vi "Controle_Manip_Main_GUI_WorkingBackup_211222.vi"() -> ()   [LabVIEW 2019] (continued)
                n3174 = local read "ESP 301 On?"() -> (w3865:bool)
                n3175 = case shown="True" w3865 {
                  tunnel: w3867 -> [_ w3881]
                  tunnel: w3866 -> [_ w3869]
                  frame False {
                  }
                  frame True {
                    n3176 = case shown="\"RotStage Exc Angle (°)\", Default" w3881 {
                      tunnel: [2 1 3] -> w3882
                      tunnel: [w3886 w3889 w3892] -> w3878
                      tunnel: w3869 -> [w3885 w3888 w3891]
                      frame "RotStage Det Angle (°)" {
                        n3177 = local write "RotStage Det Angle (°)"(w3885) -> ()
                        n3178 = control-ref of="RotStage Det Angle Readout (°)"() -> (w3886:refnum<vi>)
                      }
                      frame "Newport Linear Translation Stage Position (mm)" {
                        n3179 = control-ref of="Newport Linear Translation Stage Position Readout (mm)"() -> (w3889:refnum<vi>)
                        n3180 = local write "Newport Linear Translation Stage Position (mm)"(w3888) -> ()
                      }
                      frame "RotStage Exc Angle (°)", Default {
                        n3181 = local write "RotStage Exc Angle (°)"(w3891) -> ()
                        n3182 = control-ref of="RotStage Exc Angle Readout (°)"() -> (w3892:refnum<vi>)
                      }
                    }
                    n3183 = local read "Excitation Wavelength (nm)"() -> (w3874:dbl)
                    n3184 = local read "Photodiode handle out"() -> (w3876:refnum<visa-resource-name>)
                    n3185 = local read "Photodiode error out"() -> (w3875:errorcluster)
                    n3186 = local read "Photodiode Status"() -> (w3868:bool)
                    n3187 = local read "ESP 301 Error"() -> (w3883:errorcluster)
                    n3188 = control-ref of="Excitation Power (uW)"() -> (w3877:refnum<vi>)
                    n3189 = call <instrlib>:"TLPM Set Wavelength.vi"("error in (no error)"=w3875, "Wavelength (0.0)"=w3874, "instrument handle"=w3876) -> ("error out"=w3872:errorcluster, "instrument handle out"=w3873:refnum<visa-resource-name>)  [unwired: 7 in]
                    n3190 = local read "ESP 301 COM Port"() -> (w3884:refnum<visa-resource-name>)
                    n3191 = call "Go2Angle.vi"("VISA resource name"=w3884, "Photodiode"=w3873, "RotStage Det Angle Readout (°) 4"=w3878, "Excitation Power (uW) 2"=w3877, "Photodiode on?"=w3868, "Axis ESP301 / RotStage"=w3882, "ESP301 Error"=w3883, "Photodiode error"=w3872, "Position (units)"=w3869) -> ("Photodiode out"=w3870:refnum<visa-resource-name>, "VISA resource name out"=w3880:refnum<visa-resource-name>, "Photodiode"=w3871:errorcluster, "ESP301 Error out"=w3879:errorcluster)  [unwired: 3 in]
                    n3192 = local write "ESP 301 COM Port"(w3880) -> ()
                    n3193 = local write "ESP 301 Error"(w3879) -> ()
                    n3194 = local write "Photodiode handle out"(w3870) -> ()
                    n3195 = local write "Photodiode error out"(w3871) -> ()
                  }
                }
              }
            }
          }
          event "RotStage Exc Home", "RotStage Det Home", "Newport Linear Translation Stage Home": Mouse Down {
            n3196 = event-data() -> ("CtlRef"=w3896:refnum<vi>)  [unwired: 1 in, 7 out]
            n3197 = property class="Bool (strict)"(reference=w3896) -> ("Label.Text"=w3895:string)  [unwired: 1 in, 2 out]
            n3198 = case shown="\"Newport Linear Translation Stage Home\"" w3895 {
              tunnel: 0.0 -> [w3897 w3898 w3899]
              frame "RotStage Det Home", Default {
                n3199 = property on="RotStage Det Angle (°)" class="DigNum (strict)"("Val(Sgnl)"=w3897) -> ()  [unwired: 2 in, 2 out]
              }
              frame "Newport Linear Translation Stage Home" {
                n3200 = property on="Newport Linear Translation Stage Position (mm)" class="DigNum (strict)"("Val(Sgnl)"=w3898) -> ()  [unwired: 2 in, 2 out]
              }
              frame "RotStage Exc Home" {
                n3201 = property on="RotStage Exc Angle (°)" class="DigNum (strict)"("Val(Sgnl)"=w3899) -> ()  [unwired: 2 in, 2 out]
              }
            }
          }
          event "RotStage Exc Jog Backward", "RotStage Det Jog Backward", "RotStage Exc Jog Forward", "RotStage Det Jog Forward", "Newport Linear Translation Stage Jog Forward", "Newport Linear Translation Stage Jog Backward", "PZC Jog Forward", "PZC Jog Backward": Mouse Down {
            n3202 = event-data() -> ("CtlRef"=w3902:refnum<vi>)  [unwired: 1 in, 7 out]
            n3203 = property class="Bool (strict)"(reference=w3902) -> ("Label.Text"=w3900:string, "Value"=w3901:bool)  [unwired: 1 in, 2 out]
            n3204 = case shown="\"PZC Jog Backward\"" w3900 {
              tunnel: w3901 -> [_ _ _ _ _ _ _ _ _]
              frame "RotStage Det Jog Backward" {
                n3205 = local read "RotStage Det Angle Readout (°)"() -> (w3905:dbl)
                n3206 = local read "RotStage Det Angle Step (°)"() -> (w3904:dbl)
                n3207 = Subtract(x=w3905, y=w3904) -> (x-y=w3903:dbl)
                n3208 = property on="RotStage Det Angle (°)" class="DigNum (strict)"("Val(Sgnl)"=w3903) -> ()  [unwired: 2 in, 2 out]
              }
              frame "RotStage Det Jog Forward" {
                n3209 = local read "RotStage Det Angle Readout (°)"() -> (w3907:dbl)
                n3210 = local read "RotStage Det Angle Step (°)"() -> (w3908:dbl)
                n3211 = Add(x=w3907, y=w3908) -> (x+y=w3906:dbl)
                n3212 = property on="RotStage Det Angle (°)" class="DigNum (strict)"("Val(Sgnl)"=w3906) -> ()  [unwired: 2 in, 2 out]
              }
              frame "RotStage Exc Jog Forward" {
                n3213 = local read "RotStage Exc Angle Readout (°)"() -> (w3911:dbl)
                n3214 = local read "RotStage Exc Angle Step (°)"() -> (w3910:dbl)
                n3215 = Add(x=w3911, y=w3910) -> (x+y=w3909:dbl)
                n3216 = property on="RotStage Exc Angle (°)" class="DigNum (strict)"("Val(Sgnl)"=w3909) -> ()  [unwired: 2 in, 2 out]
              }
              frame "Newport Linear Translation Stage Jog Forward" {
                n3217 = local read "Newport Linear Translation Stage Position Readout (mm)"() -> (w3916:dbl)
                n3218 = local read "Newport Linear Translation Stage Step (mm)"() -> (w3915:dbl)
                n3219 = Add(x=w3916, y=w3915) -> (x+y=w3914:dbl)
                n3220 = property on="Newport Linear Translation Stage Position Readout (mm)" class="DigNum (strict)"() -> ("Maximum"=w3912:dbl)  [unwired: 2 in, 2 out]
                n3221 = Less Or Equal?(x=w3914, y=w3912) -> (x <= y?=w3913:bool)
                n3222 = case shown="True" w3913 {
                  tunnel: w3914 -> [_ w3920]
                  frame False {
                    n3223 = stacked-sequence {
                      frame #0 {
                        n3224 = property on="Newport Linear Translation Stage Position Readout (mm)" class="DigNum (strict)"("Blinking"=TRUE) -> ()  [unwired: 2 in, 2 out]
                      }
                      frame #1 {
                        n3225 = Wait (ms)(milliseconds to wait=u32 500) -> ()  [unwired: 1 out]
                      }
                      frame #2 {
                        n3226 = property on="Newport Linear Translation Stage Position Readout (mm)" class="DigNum (strict)"("Blinking"=FALSE) -> ()  [unwired: 2 in, 2 out]
                      }
                    }
                  }
                  frame True {
                    n3227 = property on="Newport Linear Translation Stage Position (mm)" class="DigNum (strict)"("Val(Sgnl)"=w3920) -> ()  [unwired: 2 in, 2 out]
                  }
                }
              }
              frame "Newport Linear Translation Stage Jog Backward" {
                n3228 = local read "Newport Linear Translation Stage Position Readout (mm)"() -> (w3925:dbl)
                n3229 = local read "Newport Linear Translation Stage Step (mm)"() -> (w3924:dbl)
                n3230 = Subtract(x=w3925, y=w3924) -> (x-y=w3922:dbl)
                n3231 = property on="Newport Linear Translation Stage Position Readout (mm)" class="DigNum (strict)"() -> ("Minimum"=w3921:dbl)  [unwired: 2 in, 2 out]
                n3232 = Greater Or Equal?(x=w3922, y=w3921) -> (x >= y?=w3923:bool)
                n3233 = case shown="False" w3923 {
                  tunnel: w3922 -> [_ w3929]
                  frame False {
                    n3234 = stacked-sequence {
                      frame #0 {
                        n3235 = property on="Newport Linear Translation Stage Position Readout (mm)" class="DigNum (strict)"("Blinking"=TRUE) -> ()  [unwired: 2 in, 2 out]
                      }
                      frame #1 {
                        n3236 = Wait (ms)(milliseconds to wait=u32 500) -> ()  [unwired: 1 out]
                      }
                      frame #2 {
                        n3237 = property on="Newport Linear Translation Stage Position Readout (mm)" class="DigNum (strict)"("Blinking"=FALSE) -> ()  [unwired: 2 in, 2 out]
                      }
                    }
                  }
                  frame True {
                    n3238 = property on="Newport Linear Translation Stage Position (mm)" class="DigNum (strict)"("Val(Sgnl)"=w3929) -> ()  [unwired: 2 in, 2 out]
                  }
                }
              }
              frame "RotStage Exc Jog Backward" {
                n3239 = local read "RotStage Exc Angle Readout (°)"() -> (w3932:dbl)
                n3240 = local read "RotStage Exc Angle Step (°)"() -> (w3931:dbl)
                n3241 = Subtract(x=w3932, y=w3931) -> (x-y=w3930:dbl)
                n3242 = property on="RotStage Exc Angle (°)" class="DigNum (strict)"("Val(Sgnl)"=w3930) -> ()  [unwired: 2 in, 2 out]
              }
              frame "PZC Jog Forward" {
                n3243 = local read "PZC200 Instrument Channel"() -> (w3950:string)
                n3244 = local read "PZC Speed (usteps/s)"() -> (w3941:u16)
                n3245 = Number To Decimal String(number=w3941) -> (decimal integer string=w3943:string)  [unwired: 1 in]
                n3246 = Concatenate Strings("1JA" ("Command"), w3943) -> (w3949:string)
                n3247 = call "SendCommand.vi"("Command"=w3949, "Instrument Channel"=w3950) -> ("error out"=w3947:errorcluster, "Instrument Channel out"=w3948:string)  [unwired: 8 in]
                n3248 = call "ReadCommand.vi"("Disable MAV check (F)"=FALSE, "error in"=w3947, "Instrument Channel"=w3948) -> ("error out"=w3944:errorcluster, "Instrument Channel out"=w3946:string)  [unwired: 6 in, 1 out]
                n3249 = while {
                  shift-right: [w3954] -> w3940
                  shift-left: w3946 -> [w3958]
                  shift-right: [w3952] -> w3939
                  shift-left: w3944 -> [w3953]
                  tunnel: ["1ST"] -> w3938
                  stop <- w3955 continue-if-true
                  n3250 = call "PZCGetPos.vi"("error in"=w3953, "Instrument Channel"=w3958) -> ("Instrument Channel Out"=w3954:string, "Position"=w3957:i32, "error out"=w3952:errorcluster)
                  n3251 = Wait (ms)(milliseconds to wait=u32 150) -> ()  [unwired: 1 out]
                  n3252 = local write "PZC Position Readout (usteps)"(w3957) -> ()
                  n3253 = local read "PZC Jog Forward"() -> (w3955:bool)
                }
                n3254 = call "SendCommand.vi"("error in"=w3939, "Command"=w3938, "Instrument Channel"=w3940) -> ("error out"=w3936:errorcluster, "Instrument Channel out"=w3937:string)  [unwired: 7 in]
                n3255 = call "PZCGetPos.vi"("error in"=w3936, "Instrument Channel"=w3937) -> ("Instrument Channel Out"=w3935:string, "Position"=w3933:i32, "error out"=w3934:errorcluster)
                n3256 = local write "PZC Position Readout (usteps)"(w3933) -> ()
                n3257 = local write "PZC Error"(w3934) -> ()
                n3258 = local write "PZC200 Instrument Channel"(w3935) -> ()
              }
              frame Default {
              }
              frame "PZC Jog Backward" {
                n3259 = local read "PZC Speed (usteps/s)"() -> (w3964:u16)
                n3260 = local read "PZC200 Instrument Channel"() -> (w3976:string)
                n3261 = Number To Decimal String(number=w3964) -> (decimal integer string=w3966:string)  [unwired: 1 in]
                n3262 = Concatenate Strings("1JA-" ("Command"), w3966) -> (w3975:string)
                n3263 = call "SendCommand.vi"("Command"=w3975, "Instrument Channel"=w3976) -> ("error out"=w3973:errorcluster, "Instrument Channel out"=w3974:string)  [unwired: 8 in]
                n3264 = call "ReadCommand.vi"("Disable MAV check (F)"=FALSE, "error in"=w3973, "Instrument Channel"=w3974) -> ("error out"=w3970:errorcluster, "Instrument Channel out"=w3971:string)  [unwired: 6 in, 1 out]
                n3265 = while {
                  shift-right: [w3978] -> w3969
                  shift-left: w3970 -> [w3979]
                  shift-right: [w3980] -> w3968
                  shift-left: w3971 -> [w3984]
                  tunnel: ["1ST"] -> w3967
                  stop <- w3982 continue-if-true
                  n3266 = call "PZCGetPos.vi"("error in"=w3979, "Instrument Channel"=w3984) -> ("Instrument Channel Out"=w3980:string, "Position"=w3983:i32, "error out"=w3978:errorcluster)
                  n3267 = Wait (ms)(milliseconds to wait=u32 150) -> ()  [unwired: 1 out]
                  n3268 = local write "PZC Position Readout (usteps)"(w3983) -> ()
                  n3269 = local read "PZC Jog Backward"() -> (w3982:bool)
                }
                n3270 = call "SendCommand.vi"("error in"=w3969, "Command"=w3967, "Instrument Channel"=w3968) -> ("error out"=w3963:errorcluster, "Instrument Channel out"=w3962:string)  [unwired: 7 in]
                n3271 = call "PZCGetPos.vi"("error in"=w3963, "Instrument Channel"=w3962) -> ("Instrument Channel Out"=w3961:string, "Position"=w3959:i32, "error out"=w3960:errorcluster)
                n3272 = local write "PZC Position Readout (usteps)"(w3959) -> ()
                n3273 = local write "PZC Error"(w3960) -> ()
                n3274 = local write "PZC200 Instrument Channel"(w3961) -> ()
              }
            }
          }
          event "RotStage Exc Velocity (°/s)", "RotStage Det Velocity (°/s)", "Newport Linear Translation Stage Velocity (mm/s)": Value Change {
            n3275 = event-data() -> ("CtlRef"=w3987:refnum<vi>, "NewVal"=w3986:dbl)  [unwired: 1 in, 4 out]
            n3276 = local read "ESP 301 On?"() -> (w3985:bool)
            n3277 = case shown="True" w3985 {
              tunnel: w3987 -> [_ w3994]
              tunnel: w3986 -> [_ w3992]
              frame False {
              }
              frame True {
                n3278 = local read "ESP 301 COM Port"() -> (w3991:refnum<visa-resource-name>)
                n3279 = property class="DigNum (strict)"(reference=w3994) -> ("Label.Text"=w3993:string)  [unwired: 1 in, 2 out]
                n3280 = local read "ESP 301 Error"() -> (w3990:errorcluster)
                n3281 = case shown="\"RotStage Det Velocity (°/s)\"" w3993 {
                  tunnel: w3992 -> [w3998 _ w4003 w4013]
                  tunnel: w3991 -> [w3999 w4002 w4005 w4012]
                  tunnel: w3990 -> [w4000 w4001 w4006 w4011]
                  tunnel: [w3996 w4002 w4008 w4010] -> w3989
                  tunnel: [w3995 w4001 w4007 w4009] -> w3988
                  frame "Newport Linear Translation Stage Velocity (mm/s)" {
                    n3282 = call "Set Velocity.vi"("error in (no error)"=w4000, "Velocity (units/s)"=w3998, "Axis (1)"=1, "VISA resource name"=w3999) -> ("error out"=w3995:errorcluster, "VISA resource name out"=w3996:refnum<visa-resource-name>)  [unwired: 2 in]
                  }
                  frame Default {
                  }
                  frame "RotStage Det Velocity (°/s)" {
                    n3283 = call "Set Velocity.vi"("error in (no error)"=w4006, "Velocity (units/s)"=w4003, "Axis (1)"=2, "VISA resource name"=w4005) -> ("error out"=w4007:errorcluster, "VISA resource name out"=w4008:refnum<visa-resource-name>)  [unwired: 2 in]
                  }
                  frame "RotStage Exc Velocity (°/s)" {
                    n3284 = call "Set Velocity.vi"("error in (no error)"=w4011, "Velocity (units/s)"=w4013, "Axis (1)"=3, "VISA resource name"=w4012) -> ("error out"=w4009:errorcluster, "VISA resource name out"=w4010:refnum<visa-resource-name>)  [unwired: 2 in]
                  }
                }
                n3285 = local write "ESP 301 COM Port"(w3989) -> ()
                n3286 = local write "ESP 301 Error"(w3988) -> ()
              }
            }
          }
          event "Save Spectrum", "Save Spectrum N", "Save XY Map", "Save Polarisation", "Save Contrast", "Save Michelson", "Save Custom Diode Spectrum", "Save fPow", "Save PLE": Value Change {
            n3287 = event-data() -> ("CtlRef"=w4022:refnum<vi>)  [unwired: 1 in, 3 out]
            n3288 = property class="Bool (strict)"(reference=w4022) -> ("Label.Text"=w4021:string)  [unwired: 1 in, 2 out]
            n3289 = stacked-sequence {
              tunnel: w4021 -> [_ w4071 _]
              tunnel: [_ w4068 _] -> w4019
              tunnel: [_ w4070 _] -> w4020
              tunnel: [_ w4065 _] -> w4017
              tunnel: [w4023 _ _] -> w4016
              tunnel: [_ w4066 _] -> w4018
              frame #0 {
                n3290 = local read "Excitation Wavelength (nm)"() -> (w4045:dbl)
                n3291 = local read "Wavelength calibration"() -> (w4046:dbl[])
                n3292 = local read "Center Wavelength (nm)"() -> (w4054:dbl)
                n3293 = local read "Experiment Name With Date"() -> (w4050:string)
                n3294 = local read "Map Marker Y Pos"() -> (w4036:i8)
                n3295 = local read "Scan Y Readout (V)"() -> (w4034:dbl)
                n3296 = local read "Scan X Readout (V)"() -> (w4035:dbl)
                n3297 = local read "Exposure Time (ms)"() -> (w4047:dbl)
                n3298 = local read "Map Marker X Pos"() -> (w4037:i8)
                n3299 = local read "Exposure Time (ms)"() -> (w4051:dbl)
                n3300 = local read "Attocubes On?"() -> (w4041:bool)
                n3301 = local read "Excitation Source"() -> (w4052:enum16{"P", "CW", "SK"})
                n3302 = local read "Temperature (K)"() -> (w4055:dbl)
                n3303 = local read "Excitation Power (uW)"() -> (w4057:dbl)
                n3304 = local read "Comment"() -> (w4056:string)
                n3305 = local read "Acq Mode"() -> (w4049:T3)
                n3306 = local read "Log file"() -> (w4048:string)
                n3307 = case shown="True" w4041 {
                  tunnel: [w4058 w4061] -> w4040
                  tunnel: [w4058 w4060] -> w4039
                  tunnel: [w4058 w4059] -> w4038
                  frame False {
                    w4058 = nan
                  }
                  frame True {
                    n3308 = local read "Att Pos Y"() -> (w4060:dbl)
                    n3309 = local read "Att Pos X"() -> (w4061:dbl)
                    n3310 = local read "Att Pos Z"() -> (w4059:dbl)
                  }
                }
                n3311 = Multiply(x=w4057, y=1000000.0) -> (x*y=w4053:dbl)
                n3312 = local read "LightField On?"() -> (w4043:bool)
                n3313 = Bundle("Att Pos X"=w4040, "Att Pos Y"=w4039, "Att Pos Z"=w4038, "Map Marker X Pos"=w4037, "Map Marker Y Pos"=w4036, "Scan X Readout (V)"=w4035, "Scan Y Readout (V)"=w4034) -> (w4033:T5)  [unwired: 1 in]
                "Location cluster" <- w4033
                n3314 = case shown="False" w4043 {
                  tunnel: ["" w4063] -> w4042
                  frame False {
                  }
                  frame True {
                    n3315 = local read "Grating"() -> (w4063:string)
                  }
                }
                n3316 = Bundle("Sample first cooldown"="Sample first cooldown", "SampleOf"="SampleOf", "Synthesis/Name"="Synthesis/Name", "Synthesis/InjTemp"="Synthesis/InjTemp", "Synthesis/Dilution"="Synthesis/Dilution", "Synthesis/Polymer"="Synthesis/Polymer", "Synthesis/DilutionPolyRatio"="Synthesis/DilutionPolyRatio", "Synthesis/Solvent"="Synthesis/Solvent") -> (w4024:T40)  [unwired: 1 in]
                n3317 = Bundle("Comment"=w4056, "Temperature (K)"=w4055, "Center Wavelength (nm)"=w4054, w4053, "Excitation Source"=w4052, "Exposure Time (ms)"=w4051, "Experiment Name With Date"=w4050, "Acq Mode"=w4049, "Log file"=w4048, "Exposure Time (ms)"=w4047, "Wavelength calibration"=w4046, "Excitation Wavelength (nm)"=w4045, "Grating"=w4042, w4033, w4024) -> (w4023:T41)  [unwired: 1 in]
                "Params Save" <- w4023
              }
              frame #1 {
                n3318 = case shown="\"Save Contrast\"" w4071 {
                  tunnel: [w4075 w4120 w4145 w4169 w4191 w4221 w4244 w4267 w4316] -> w4068
                  tunnel: [w4074 w4118 w4144 w4168 w4190 w4220 w4243 w4266 w4313] -> w4065
                  tunnel: [w4073 w4119 w4143 w4167 w4189 w4219 w4242 w4265 w4307] -> w4069
                  tunnel: [w4072 w4117 w4142 w4166 w4188 w4218 w4241 w4264 w4306] -> w4066
                  frame "Save Spectrum N" {
                    n3319 = local read "Acq Mode"() -> (w4076:T3)
                    n3320 = case shown="\"Spectrum\", Default" w4076 {
                      tunnel: [w4085 w4106] -> w4075
                      tunnel: [w4084 w4105] -> w4074
                      tunnel: [w4078 w4099] -> w4073
                      tunnel: [w4077 w4098] -> w4072
                      frame "Spectrum", Default {
                        w4077 = T42."Time Trace" ("Measurement type")
                        n3321 = invoke on="CCD 2D Image Main" class="IntGraph (strict)" method="Get Image"() -> ("image data"=w4078:T43)  [unwired: 6 in, 5 out]
                        n3322 = local read "BackgroundSpec"() -> (w4082:dbl[])
                        n3323 = local read "Pol in path?"() -> (w4081:bool)
                        n3324 = local read "DotNum"() -> (w4083:dbl)
                        n3325 = local read "Data"() -> (w4091:T26)
                        n3326 = local read "Params Save"() -> (w4094:T4)
                        n3327 = Index Array(array=w4091, index=0) -> (element=w4089:T44)
                        n3328 = case shown="True" w4081 {
                          tunnel: [w4095 w4096] -> w4079
                          tunnel: [w4095 w4097] -> w4080
                          frame False {
                            w4095 = nan
                          }
                          frame True {
                            n3329 = local read "RotStage Exc Angle Readout (°)"() -> (w4097:dbl)
                            n3330 = local read "RotStage Det Angle Readout (°)"() -> (w4096:dbl)
                          }
                        }
                        n3331 = Unbundle By Name(w4089) -> ("Image"=w4088:dbl[][][])
                        "Image" <- w4088
                        n3332 = Index Array(array=w4088, index (dim 1)=0 ("disabled index (row)")) -> (element=w4087:dbl[][])  [unwired: 2 in]
                        n3333 = Build Array(w4080) -> (w4093:dbl[])
                        n3334 = Build Array(w4079) -> (w4092:dbl[])
                        n3335 = call "Format&SaveDataCleanbckp.vi"("Measurement type"=w4077, "Params Save"=w4094, "DotNum"=w4083, "Suppl"=w4082, "Data_CCD_px"=w4087, "L2Exc_deg"=w4093, "L2Det_deg"=w4092) -> ("FullComment"=w4084:string, "WrittenDatasetName"=w4085:string)  [unwired: 9 in, 2 out]
                      }
                      frame "Image" {
                        w4098 = T42."Time Trace" ("Measurement type")
                        n3336 = invoke on="CCD 2D Image Main" class="IntGraph (strict)" method="Get Image"() -> ("image data"=w4099:T43)  [unwired: 6 in, 5 out]
                        n3337 = local read "BackgroundSpec"() -> (w4103:dbl[])
                        n3338 = local read "Pol in path?"() -> (w4102:bool)
                        n3339 = local read "DotNum"() -> (w4104:dbl)
                        n3340 = local read "Data"() -> (w4110:T26)
                        n3341 = local read "Params Save"() -> (w4113:T4)
                        n3342 = case shown="True" w4102 {
                          tunnel: [w4114 w4115] -> w4100
                          tunnel: [w4114 w4116] -> w4101
                          frame False {
                            w4114 = nan
                          }
                          frame True {
                            n3343 = local read "RotStage Exc Angle Readout (°)"() -> (w4116:dbl)
                            n3344 = local read "RotStage Det Angle Readout (°)"() -> (w4115:dbl)
                          }
                        }
                        n3345 = Index Array(array=w4110, index=0) -> (element=w4108:T44)
                        n3346 = Unbundle By Name(w4108) -> ("Image"=w4107:dbl[][][])
                        n3347 = Build Array(w4101) -> (w4112:dbl[])
                        n3348 = Build Array(w4100) -> (w4111:dbl[])
                        n3349 = call "Format&SaveDataCleanbckp.vi"("Measurement type"=w4098, "Params Save"=w4113, "DotNum"=w4104, "Main 3D Data to write"=w4107, "Suppl"=w4103, "L2Exc_deg"=w4112, "L2Det_deg"=w4111) -> ("FullComment"=w4105:string, "WrittenDatasetName"=w4106:string)  [unwired: 9 in, 2 out]
                      }
                    }
                  }
                  frame "Save XY Map" {
                    w4117 = T42."XY Intensity Map" ("Measurement type")
                    n3350 = local read "Pol in path?"() -> (w4131:bool)
                    n3351 = local read "Params Save"() -> (w4138:T4)
                    n3352 = local read "BackgroundSpec"() -> (w4135:dbl[])
                    n3353 = local read "Params XY Map SubVI"() -> (w4128:T23)
                    n3354 = local read "Map Marker Y Pos"() -> (w4126:i8)
                    n3355 = local read "XYMap Data"() -> (w4137:i32[][])
                    n3356 = local read "Map Marker X Pos"() -> (w4127:i8)
                    n3357 = local read "XYPositions"() -> (w4134:dbl[][])
                    n3358 = Format Into String(w4127) -> (resulting string=w4125:string)  [unwired: 3 in, 1 out]
                    n3359 = Format Into String(w4126) -> (resulting string=w4124:string)  [unwired: 3 in, 1 out]
                    n3360 = case shown="True" w4131 {
                      tunnel: [w4139 w4140] -> w4130
                      tunnel: [w4139 w4141] -> w4129
                      frame False {
                        w4139 = nan
                      }
                      frame True {
                        n3361 = local read "RotStage Exc Angle Readout (°)"() -> (w4141:dbl)
                        n3362 = local read "RotStage Det Angle Readout (°)"() -> (w4140:dbl)
                      }
                    }
                    n3363 = Concatenate Strings("\n### Map @ " ("string"), w4125, "x" ("string"), w4124) -> (w4123:string)
                    n3364 = call "Write2Markdown.vi"("String"=w4123) -> ()
                    n3365 = disable-structure shown="Disabled" {
                      frame Disabled {
                        n3366 = local read "XYPos Indices"() -> ()  [unwired: 1 out]
                      }
                      frame Enabled {
                      }
                    }
                    n3367 = Build Array(w4130) -> (w4133:dbl[])
                    n3368 = Build Array(w4129) -> (w4132:dbl[])
                    n3369 = call "Format&SaveDataCleanbckp.vi"("Measurement type"=w4117, "Suppl_2D"=w4134, "Params Save"=w4138, "DotNum"=0.0, "Params XY Map SubVI"=w4128, "Suppl"=w4135, "Data_CCD_px"=w4137, "L2Exc_deg"=w4132, "L2Det_deg"=w4133) -> ("FullComment"=w4118:string, "WrittenDatasetName"=w4120:string)  [unwired: 7 in, 2 out]
                    n3370 = invoke on="XY Intensity Map" class="IntGraph (strict)" method="Get Image"() -> ("image data"=w4119:T43)  [unwired: 6 in, 5 out]
                  }
                  frame "Save Contrast" {
                    n3371 = local read "Acq Mode"() -> (w4146:T3)
                    n3372 = case shown="\"Spectrum\", Default" w4146 {
                      tunnel: [w4156] -> w4145
                      tunnel: [w4155] -> w4144
                      tunnel: [w4149] -> w4143
                      tunnel: [w4148] -> _
                      tunnel: [w4147] -> w4142
                      frame "Spectrum", Default {
                        w4147 = T42."Contrast" ("Measurement type")
                        n3373 = invoke on="Contrast Oscillations" class="XYGraph (strict)" method="Get Image"() -> ("image data"=w4149:T43)  [unwired: 6 in, 5 out]
                        n3374 = local read "Pol in path?"() -> (w4152:bool)
                        n3375 = local read "BackgroundSpec"() -> (w4153:dbl[])
                        n3376 = local read "DotNum"() -> (w4154:dbl)
                        n3377 = local read "Params Save"() -> (w4162:T4)
                        n3378 = case shown="True" w4152 {
                          tunnel: [w4163 w4164] -> w4150
                          tunnel: [w4163 w4165] -> w4151
                          frame False {
                            w4163 = nan
                          }
                          frame True {
                            n3379 = local read "RotStage Exc Angle Readout (°)"() -> (w4165:dbl)
                            n3380 = local read "RotStage Det Angle Readout (°)"() -> (w4164:dbl)
                          }
                        }
                        n3381 = local read "Contrast Array Out"() -> (w4159:dbl[][])
                        n3382 = local read "PZAPos&Pow"() -> (w4157:dbl[][])
                        n3383 = Build Array(w4151) -> (w4161:dbl[])
                        n3384 = Build Array(w4150) -> (w4160:dbl[])
                        n3385 = Transpose 2D Array(2D array=w4159) -> (transposed array=w4158:dbl[][])
                        n3386 = call "Format&SaveDataCleanbckp.vi"("Measurement type"=w4147, "Suppl_2D"=w4157, "Params Save"=w4162, "DotNum"=w4154, "Suppl"=w4153, "Data_CCD_px"=w4158, "L2Exc_deg"=w4161, "L2Det_deg"=w4160) -> ("datasetnumber"=w4148:string, "FullComment"=w4155:string, "WrittenDatasetName"=w4156:string)  [unwired: 8 in, 1 out]
                      }
                    }
                  }
                  frame "Save Michelson" {
                    n3387 = local read "Acq Mode"() -> (w4170:T3)
                    n3388 = case shown="\"Spectrum\", Default" w4170 {
                      tunnel: [w4179] -> w4169
                      tunnel: [w4178] -> w4168
                      tunnel: [w4172] -> w4167
                      tunnel: [w4171] -> w4166
                      frame "Spectrum", Default {
                        w4171 = T42."Michelson" ("Measurement type")
                        n3389 = local read "BackgroundSpec"() -> (w4176:dbl[])
                        n3390 = invoke on="Contrast Oscillations" class="XYGraph (strict)" method="Get Image"() -> ("image data"=w4172:T43)  [unwired: 6 in, 5 out]
                        n3391 = local read "Pol in path?"() -> (w4175:bool)
                        n3392 = local read "DotNum"() -> (w4177:dbl)
                        n3393 = local read "Params Save"() -> (w4184:T4)
                        n3394 = case shown="True" w4175 {
                          tunnel: [w4185 w4186] -> w4173
                          tunnel: [w4185 w4187] -> w4174
                          frame False {
                            w4185 = nan
                          }
                          frame True {
                            n3395 = local read "RotStage Exc Angle Readout (°)"() -> (w4187:dbl)
                            n3396 = local read "RotStage Det Angle Readout (°)"() -> (w4186:dbl)
                          }
                        }
                        n3397 = local read "Michelson Array Out"() -> (w4180:dbl[][][])
                        n3398 = local read "PZC&Pow3D"() -> (w4181:dbl[][][])
                        n3399 = Build Array(w4174) -> (w4183:dbl[])
                        n3400 = Build Array(w4173) -> (w4182:dbl[])
                        n3401 = call "Format&SaveDataCleanbckp.vi"("Measurement type"=w4171, "Params Save"=w4184, "DotNum"=w4177, "Main 3D Data to write"=w4180, "Suppl"=w4176, "L2Exc_deg"=w4183, "L2Det_deg"=w4182, "Suppl_3D"=w4181) -> ("FullComment"=w4178:string, "WrittenDatasetName"=w4179:string)  [unwired: 8 in, 2 out]
                      }
                    }
                  }
                  frame "Save Polarisation" {
                    n3402 = local read "Acq Mode"() -> (w4192:T3)
                    n3403 = case shown="\"Spectrum\", Default" w4192 {
                      tunnel: [w4202] -> w4191
                      tunnel: [w4201] -> w4190
                      tunnel: [w4195] -> w4189
                      tunnel: [w4194] -> w4188
                      frame "Spectrum", Default {
                        w4194 = T42."Polarisation" ("Measurement type")
                        n3404 = local read "Pol in path?"() -> (w4198:bool)
                        n3405 = case shown="True" w4198 {
                          tunnel: [w4205 w4208] -> w4197
                          tunnel: [w4205 w4207] -> w4196
                          frame False {
                            n3406 = Build Array(nan) -> (w4205:dbl[])
                          }
                          frame True {
                            n3407 = local read "Polar mode"() -> (w4209:u16)
                            n3408 = case shown="3, Default" w4209 {
                              tunnel: [w4211 w4213] -> w4208
                              tunnel: [w4210 w4216] -> w4207
                              frame 2 {
                                n3409 = local read "RotStage Exc Angle Readout (°)"() -> (w4212:dbl)
                                n3410 = local read "Angles"() -> (w4210:dbl[])
                                n3411 = Build Array(w4212) -> (w4211:dbl[])
                              }
                              frame 3, Default {
                                n3412 = local read "PuissancesPolar"() -> (w4214:dbl[])
                                n3413 = local read "Angles"() -> (w4215:dbl[])
                                n3414 = local read "RotStage Det Angle Readout (°)"() -> (w4217:dbl)
                                n3415 = Insert Into Array(array=w4215, new element=w4214) -> (w4213:dbl[])  [unwired: 1 in]
                                n3416 = Build Array(w4217) -> (w4216:dbl[])
                              }
                            }
                          }
                        }
                        n3417 = local read "PuissancesPolar"() -> (w4193:dbl[])
                        n3418 = local read "BackgroundSpec"() -> (w4199:dbl[])
                        n3419 = local read "Params Save"() -> (w4204:T4)
                        n3420 = local read "DotNum"() -> (w4200:dbl)
                        n3421 = invoke on="Polarisation 2D Image" class="IntGraph (strict)" method="Get Image"() -> ("image data"=w4195:T43)  [unwired: 6 in, 5 out]
                        n3422 = property on="Polarisation 2D Image" class="IntGraph (strict)"() -> ("Value"=w4203:dbl[][])  [unwired: 2 in, 2 out]
                        n3423 = call "Format&SaveDataCleanbckp.vi"("Data_Angle_deg"=w4193, "Measurement type"=w4194, "Params Save"=w4204, "DotNum"=w4200, "Suppl"=w4199, "Data_CCD_px"=w4203, "L2Exc_deg"=w4197, "L2Det_deg"=w4196) -> ("FullComment"=w4201:string, "WrittenDatasetName"=w4202:string)  [unwired: 8 in, 2 out]
                      }
                    }
                  }
                  frame "Save PLE" {
                    n3424 = local read "Acq Mode"() -> (w4222:T3)
                    n3425 = case shown="\"Spectrum\", Default" w4222 {
                      tunnel: [w4233] -> w4221
                      tunnel: [w4232] -> w4220
                      tunnel: [w4223] -> w4219
                      tunnel: [w4226] -> w4218
                      frame "Spectrum", Default {
                        w4226 = T45."PLE" ("Measurement type")
                        n3426 = local read "Pol in path?"() -> (w4230:bool)
                        n3427 = local read "PLE 2D ExcWL&Pow"() -> (w4225:dbl[][])
                        n3428 = local read "PLE Raw Intensity"() -> (w4224:i32[][])
                        n3429 = case shown="True" w4230 {
                          tunnel: [w4235 w4240] -> w4228
                          tunnel: [w4235 w4237] -> w4227
                          frame False {
                            n3430 = Build Array(nan) -> (w4235:dbl[])
                          }
                          frame True {
                            n3431 = local read "RotStage Exc Angle Readout (°)"() -> (w4239:dbl)
                            n3432 = local read "RotStage Det Angle Readout (°)"() -> (w4238:dbl)
                            n3433 = Build Array(w4239) -> (w4240:dbl[])
                            n3434 = Build Array(w4238) -> (w4237:dbl[])
                          }
                        }
                        n3435 = local read "BackgroundSpec"() -> (w4229:dbl[])
                        n3436 = local read "Params Save"() -> (w4234:T4)
                        n3437 = local read "DotNum"() -> (w4231:dbl)
                        n3438 = call "Format&SaveDataCleanbckp.vi"("Measurement type"=w4226, "Suppl_2D"=w4225, "Params Save"=w4234, "DotNum"=w4231, "Suppl"=w4229, "Data_CCD_px"=w4224, "L2Exc_deg"=w4228, "L2Det_deg"=w4227) -> ("FullComment"=w4232:string, "WrittenDatasetName"=w4233:string)  [unwired: 8 in, 2 out]
                        n3439 = invoke on="PLE Raw Intensity" class="IntGraph (strict)" method="Get Image"() -> ("image data"=w4223:T43)  [unwired: 6 in, 5 out]
                      }
                    }
                  }
                  frame "Save fPow" {
                    n3440 = local read "Acq Mode"() -> (w4245:T3)
                    n3441 = case shown="\"Spectrum\", Default" w4245 {
                      tunnel: [w4258] -> w4244
                      tunnel: [w4257] -> w4243
                      tunnel: [w4246] -> w4242
                      tunnel: [w4249] -> w4241
                      frame "Spectrum", Default {
                        w4249 = T42."fPow" ("Measurement type")
                        n3442 = local read "DotNum"() -> (w4255:dbl)
                        n3443 = local read "Pol in path?"() -> (w4252:bool)
                        n3444 = local read "Array fPow Pow"() -> (w4248:dbl[])
                        n3445 = local read "Params Save"() -> (w4253:T4)
                        n3446 = case shown="False" w4252 {
                          tunnel: [w4261 w4263] -> w4251
                          tunnel: [w4261 w4262] -> w4250
                          frame False {
                            w4261 = nan
                          }
                          frame True {
                            n3447 = local read "RotStage Exc Angle Readout (°)"() -> (w4262:dbl)
                            n3448 = local read "RotStage Det Angle Readout (°)"() -> (w4263:dbl)
                          }
                        }
                        n3449 = local read "Array fPow"() -> (w4256:i32[][])
                        n3450 = Build Array(w4248, w4248) -> (w4247:dbl[][])
                        n3451 = invoke on="CCD 2D Image Main" class="IntGraph (strict)" method="Get Image"() -> ("image data"=w4246:T43)  [unwired: 6 in, 5 out]
                        n3452 = local read "BackgroundSpec"() -> (w4254:dbl[])
                        n3453 = Build Array(w4250) -> (w4260:dbl[])
                        n3454 = Build Array(w4251) -> (w4259:dbl[])
                        n3455 = call "Format&SaveDataCleanbckp.vi"("Measurement type"=w4249, "Suppl_2D"=w4247, "Params Save"=w4253, "DotNum"=w4255, "Suppl"=w4254, "Data_CCD_px"=w4256, "L2Exc_deg"=w4260, "L2Det_deg"=w4259) -> ("FullComment"=w4257:string, "WrittenDatasetName"=w4258:string)  [unwired: 8 in, 2 out]
                      }
                    }
                  }
                  frame "Save Spectrum", Default {
                    n3456 = local read "Acq Mode"() -> (w4268:T3)
                    n3457 = case shown="\"Spectrum\", Default" w4268 {
                      tunnel: [w4277 w4289] -> w4267
                      tunnel: [w4276 w4296] -> w4266
                      tunnel: [w4270 w4290] -> w4265
                      tunnel: [w4269 w4288] -> w4264
                      frame "Spectrum", Default {
                        w4269 = T42."Spectrum" ("Measurement type")
                        n3458 = local read "Pol in path?"() -> (w4273:bool)
                        n3459 = invoke on="CCD 1D Spectrum Main" class="XYGraph (strict)" method="Get Image"() -> ("image data"=w4270:T43)  [unwired: 6 in, 5 out]
                        n3460 = local read "CCD 1D Spectrum Main"() -> (w4281:cluster{dbl[], dbl[]})
                        n3461 = local read "DotNum"() -> (w4275:dbl)
                        n3462 = local read "BackgroundSpec"() -> (w4274:dbl[])
                        n3463 = local read "Params Save"() -> (w4284:T4)
                        n3464 = case shown="True" w4273 {
                          tunnel: [w4285 w4286] -> w4271
                          tunnel: [w4285 w4287] -> w4272
                          frame False {
                            w4285 = nan
                          }
                          frame True {
                            n3465 = local read "RotStage Exc Angle Readout (°)"() -> (w4287:dbl)
                            n3466 = local read "RotStage Det Angle Readout (°)"() -> (w4286:dbl)
                          }
                        }
                        n3467 = Unbundle(w4281) -> (w4280:dbl[], w4279:dbl[])
                        n3468 = Build Array(w4272) -> (w4283:dbl[])
                        n3469 = Build Array(w4271) -> (w4282:dbl[])
                        n3470 = Build Array(w4280, w4279) -> (w4278:dbl[][])
                        n3471 = call "Format&SaveDataCleanbckp.vi"("Measurement type"=w4269, "Params Save"=w4284, "DotNum"=w4275, "Suppl"=w4274, "Data_CCD_px"=w4278, "L2Exc_deg"=w4283, "L2Det_deg"=w4282) -> ("FullComment"=w4276:string, "WrittenDatasetName"=w4277:string)  [unwired: 9 in, 2 out]
                      }
                      frame "Image" {
                        w4288 = T42."Spectrum" ("Measurement type")
                        n3472 = invoke on="CCD 2D Image Main" class="IntGraph (strict)" method="Get Image"() -> ("image data"=w4290:T43)  [unwired: 6 in, 5 out]
                        n3473 = local read "BackgroundSpec"() -> (w4294:dbl[])
                        n3474 = local read "Pol in path?"() -> (w4293:bool)
                        n3475 = local read "DotNum"() -> (w4295:dbl)
                        n3476 = local read "Data"() -> (w4299:T26)
                        n3477 = case shown="True" w4293 {
                          tunnel: [w4303 w4304] -> w4291
                          tunnel: [w4303 w4305] -> w4292
                          frame False {
                            w4303 = nan
                          }
                          frame True {
                            n3478 = local read "RotStage Exc Angle Readout (°)"() -> (w4305:dbl)
                            n3479 = local read "RotStage Det Angle Readout (°)"() -> (w4304:dbl)
                          }
                        }
                        n3480 = Index Array(array=w4299) -> (element=w4298:T44)  [unwired: 1 in]
                        n3481 = Unbundle By Name(w4298) -> ("Image"=w4297:dbl[][][])
                        n3482 = local read "Params Save"() -> (w4302:T4)
                        n3483 = Build Array(w4292) -> (w4301:dbl[])
                        n3484 = Build Array(w4291) -> (w4300:dbl[])
                        n3485 = call "Format&SaveDataCleanbckp.vi"("Measurement type"=w4288, "Params Save"=w4302, "DotNum"=w4295, "Main 3D Data to write"=w4297, "Suppl"=w4294, "L2Exc_deg"=w4301, "L2Det_deg"=w4300) -> ("FullComment"=w4296:string, "WrittenDatasetName"=w4289:string)  [unwired: 9 in, 2 out]
                      }
                    }
                  }
                  frame "Save Custom Diode Spectrum" {
                    w4306 = T42."Spectrum" ("Measurement type")
                    n3486 = local read "Spectrum Custom Mode"() -> (w4312:u16)
                    n3487 = local read "Data PL Custom Diode Spectrum"() -> (w4319:dbl[])
                    n3488 = local read "DotNum"() -> (w4311:dbl)
                    n3489 = local read "Params Save"() -> (w4320:T4)
                    n3490 = local read "Pol in path?"() -> (w4310:bool)
                    n3491 = invoke on="CCD 1D Spectrum Main" class="XYGraph (strict)" method="Get Image"() -> ("image data"=w4307:T43)  [unwired: 6 in, 5 out]
                    n3492 = local read "Wavelength calibration"() -> (w4318:dbl[])
                    n3493 = case shown="True" w4310 {
                      tunnel: [w4321 w4322] -> w4308
                      tunnel: [w4321 w4323] -> w4309
                      frame False {
                        w4321 = nan
                      }
                      frame True {
                        n3494 = local read "RotStage Exc Angle Readout (°)"() -> (w4323:dbl)
                        n3495 = local read "RotStage Det Angle Readout (°)"() -> (w4322:dbl)
                      }
                    }
                    n3496 = Build Array(w4318, w4319) -> (w4317:dbl[][])
                    n3497 = Build Array(w4309) -> (w4315:dbl[])
                    n3498 = Build Array(w4308) -> (w4314:dbl[])
                    n3499 = call "Format&SaveDataCleanbckp.vi"("Measurement type"=w4306, "Spectrum Custom Mode"=w4312, "Params Save"=w4320, "DotNum"=w4311, "Data_CCD_px"=w4317, "L2Exc_deg"=w4315, "L2Det_deg"=w4314) -> ("FullComment"=w4313:string, "WrittenDatasetName"=w4316:string)  [unwired: 9 in, 2 out]
                  }
                }
                "WrittenDatasetName" <- w4068
                "FullComment" <- w4065
                n3500 = local read "Params Save"() -> (w4064:T4)
                n3501 = call "AutoScreenShot.vi"("Params Save"=w4064, "Figure image data"=w4069, "Datasetname"=w4068) -> ("imagefilename"=→"imagefilename":string)  [unwired: 1 in]
                n3502 = local read "Log file"() -> (w4070:string)
              }
              frame #2 {
                w4326 = FALSE
                n3503 = local write "Comment"("") -> ()
                n3504 = local write "Save Custom Diode Spectrum"(w4326) -> ()
                n3505 = local write "Save Michelson"(w4326) -> ()
                n3506 = local write "Save Contrast"(w4326) -> ()
                n3507 = local write "Save XY Map"(w4326) -> ()
                n3508 = local write "Save Spectrum"(w4326) -> ()
                n3509 = local write "Save Polarisation"(w4326) -> ()
                n3510 = local write "Save Spectrum N"(w4326) -> ()
                n3511 = local write "Save fPow"(w4326) -> ()
                n3512 = local read "DotNum"() -> (→"LastDotNum":dbl)
              }
            }
            n3513 = call "WriteSave2MarkdownWithImages.vi"("Measurement type"=w4018, "Full Comment"=w4017, "Params Save"=w4016, "Written Dataset Name"=w4019, "Log file"=w4020) -> ("Log file after"=w4015:string)  [unwired: 1 in]
            n3514 = local write "Log file"(w4015) -> ()
          }
          event "Connect": Value Change {
            n3515 = event-data() -> ("NewVal"=w4327:bool)  [unwired: 1 in, 5 out]
            n3516 = case shown="False" w4327 {
              frame False {
                n3517 = local read "PH_Init_Data"() -> (w4330:T11)
                n3518 = Unbundle By Name(w4330) -> ("Deviceindex"=w4329:i32)
                n3519 = local write "Connected"(FALSE) -> ()
                n3520 = call "PH_Close.vi"("devidx"=w4329) -> ()
              }
              frame True {
                n3521 = local read "PicoHarp On?"() -> (w4331:bool)
                n3522 = case shown="True" w4331 {
                  frame False {
                  }
                  frame True {
                    n3523 = local read "Log file"() -> (w4333:string)
                    n3524 = property on="Experiment Graph Controls" class="TabCtl (strict)"("Value"=T25."APDs" ("Experiment Graph Controls")) -> ("Pages"=w4338:refnum<vi>[])  [unwired: 2 in, 2 out]
                    n3525 = call "Write2LogFile.vi"("Add to log file"="Initialise communication with PicoHarp", "Log file before"=w4333, "Checkbox"=FALSE) -> ("Log file after"=w4334:string)
                    n3526 = call "PH_Init.vi"() -> ("PH_Init_Data"=w4332:T11)
                    n3527 = local write "Log file"(w4334) -> ()
                    n3528 = Index Array(array=w4338, index=4) -> (element=w4337:refnum<vi>)
                    n3529 = property class="Page"(reference=w4337, "PageVis"=TRUE ("Page Visible")) -> ()  [unwired: 1 in, 2 out]
                    n3530 = local write "PH_Init_Data"(w4332) -> ()
                    n3531 = local write "Connected"(TRUE) -> ()
                  }
                }
              }
            }
          }
          event "ChangeSample": Mouse Down {
            n3532 = event-data() -> ()  [unwired: 1 in, 8 out]
            n3533 = local read "Synthesis/DilutionPolyRatio"() -> (w4353:dbl)
            n3534 = local read "Synthesis/Polymer"() -> (w4356:string)
            n3535 = local read "Synthesis/Solvent"() -> (w4355:string)
            n3536 = local read "Sample first cooldown"() -> (w4357:timestamp)
            n3537 = local read "Synthesis/Dilution"() -> (w4352:dbl)
            n3538 = local read "Synthesis/Name"() -> (w4354:string)
            n3539 = local read "Synthesis/Name"() -> (w4351:string)
            n3540 = local read "Synthesis/InjTemp"() -> (w4350:dbl)
            n3541 = local read "SampleOf"() -> (w4358:string)
            n3542 = local read "SampleGoal"() -> (w4348:string)
            n3543 = Bundle("Synthesis/InjTemp"=w4350, "Synthesis/Name"=w4351, "Synthesis/Dilution"=w4352, "Synthesis/DilutionPolyRatio"=w4353, "Synthesis/Name"=w4354, "Synthesis/Solvent"=w4355, "Synthesis/Polymer"=w4356, "Sample first cooldown"=w4357, "SampleOf"=w4358) -> (w4349:T2)  [unwired: 1 in]
            n3544 = local write "output cluster"(w4349) -> ()
            n3545 = call "SampleDetails.vi"("SampleDetailsClus"=w4349, "SampleGoal"=w4348, "Wrte to Obs"=TRUE ("NewSample in Obs"), "NewSampleDetails?"=TRUE, "Header?"=FALSE) -> ("SampleNameNoDate"=w4345:string, "SampleName"=w4346:string)
            n3546 = local write "Experiment Name"(w4345) -> ()
            n3547 = local write "Experiment Name With Date"(w4346) -> ()
          }
          event "Scan FSM Go to Cursor": Mouse Down {
            n3548 = event-data() -> ()  [unwired: 1 in, 8 out]
            n3549 = local write "Scan FSM Go to Cursor"(FALSE ("Scan FSM Go to Cursor")) -> ()
            n3550 = local read "NewDot"() -> (w4360:bool)
            n3551 = property on="XY Intensity Map" class="IntGraph (strict)"() -> ("Cursor.Cursor X"=w4361:dbl, "Cursor.Cursor Y"=w4362:dbl)  [unwired: 2 in, 2 out]
            n3552 = case shown="True" w4360 {
              frame False {
              }
              frame True {
                n3553 = local read "DotNum"() -> (w4364:dbl)
                n3554 = Increment(x=w4364) -> (x+1=w4363:dbl)
                n3555 = local write "DotNum"(w4363) -> ()
                n3556 = property on="DotNum" class="DigNum (strict)"("Val(Sgnl)"=w4363) -> ()  [unwired: 2 in, 2 out]
              }
            }
            n3557 = property on="FSM Y Axis Pos" class="DigNum (strict)"("Val(Sgnl)"=w4362) -> ()  [unwired: 2 in, 2 out]
            n3558 = property on="FSM X Axis Pos" class="DigNum (strict)"("Val(Sgnl)"=w4361) -> ()  [unwired: 2 in, 2 out]
          }
          event "DotNum": Value Change {
            w4368 = "\r"
            w4386 = "\r"
            w4374 = "%02d" ("format string")
            n3559 = event-data() -> ("NewVal"=w4376:dbl)  [unwired: 1 in, 5 out]
            n3560 = local read "Map Marker Y Pos"() -> (w4408:i8)
            n3561 = local read "Map Marker X Pos"() -> (w4409:i8)
            n3562 = Format Into String(format string=w4374, initial string="#### NC" ("String"), w4376) -> (resulting string=w4379:string)  [unwired: 1 in, 1 out]
            n3563 = local read "FSM Y Axis Pos"() -> (w4402:dbl)
            n3564 = Format Into String(w4409) -> (resulting string=w4407:string)  [unwired: 3 in, 1 out]
            n3565 = Format Into String(format string=w4374, initial string="NC", w4376) -> (resulting string=w4373:string)  [unwired: 1 in, 1 out]
            n3566 = Format Into String(w4408) -> (resulting string=w4406:string)  [unwired: 3 in, 1 out]
            n3567 = local read "FSM X Axis Pos"() -> (w4401:dbl)
            n3568 = Concatenate Strings(w4373, "_Pos" ("string")) -> (w4377:string)
            n3569 = Format Into String(format string="(%.2f,", initial string=" FSM ", w4401) -> (resulting string=w4398:string)  [unwired: 1 in, 1 out]
            n3570 = Format Into String(format string="%.2f)", w4402) -> (resulting string=w4396:string)  [unwired: 2 in, 1 out]
            n3571 = flat-sequence {
              tunnel: w4370 -> [w4417]
              tunnel: w4372 -> [w4420]
              tunnel: w4371 -> [w4419]
              tunnel: [w4418] -> w4365
              tunnel: w4366 -> [w4423]
              frame #0 {
                n3572 = call "Write2Markdown.vi"("String"=w4417) -> ()
              }
              frame #1 {
                n3573 = local read "ExportMapPosition?"() -> (w4418:bool)
                n3574 = case shown="True" w4418 {
                  tunnel: w4420 -> [_ w4422]
                  tunnel: w4419 -> [_ w4421]
                  frame False {
                  }
                  frame True {
                    n3575 = call <vilib>:"Write PNG File.vi"("image data"=w4422, "path to PNG file"=w4421) -> ()  [unwired: 8 in, 2 out]
                  }
                }
              }
              frame #2 {
                n3576 = call "Write2Markdown.vi"("String"=w4423) -> ()
              }
            }
            n3577 = Concatenate Strings("\r", w4379, " @ " ("string"), w4407, "x" ("string"), w4406, w4398, "  " ("string"), w4396, w4386, "##### Position" ("string"), w4386) -> (w4370:string)
            n3578 = invoke on="XY Intensity Map" class="IntGraph (strict)" method="Get Image"() -> ("image data"=w4372:T43)  [unwired: 6 in, 5 out]
            n3579 = Format Date/Time String(time format string (%c)="\\%Y-%m-%d_") -> (date/time string=w4392:string)  [unwired: 2 in]
            n3580 = Concatenate Strings(w4392, w4377, ".png" ("string")) -> (w4393:string)
            n3581 = Concatenate Strings("C:\\Users\\manip\\Documents\\CARODOT_Data\\doc\\CARODOC\\attachments", w4393) -> (w4391:string)
            n3582 = String To Path(string=w4391) -> (path=w4371:path)
            n3583 = Format Date/Time String(time format string (%c)="%Y-%m-%d_") -> (date/time string=w4385:string)  [unwired: 2 in]
            n3584 = Concatenate Strings(w4385, w4377, ".png" ("string")) -> (w4384:string)
            n3585 = Concatenate Strings("> ![\\|300](attachments/", w4384, ")", w4368) -> (w4367:string)
            n3586 = case shown="False" w4365 {
              tunnel: "##### Measurements" ("string") -> [w4412 w4416]
              tunnel: w4368 -> [w4411 w4415]
              tunnel: w4367 -> [_ w4414]
              tunnel: [w4410 w4413] -> w4366
              frame False {
                n3587 = Concatenate Strings(w4412, w4411) -> (w4410:string)
              }
              frame True {
                n3588 = Concatenate Strings(w4414, w4416, w4415) -> (w4413:string)
              }
            }
          }
          event "Scan FSM Set as Center": Value Change {
            n3589 = event-data() -> ("CtlRef"=w4437:refnum<vi>)  [unwired: 1 in, 5 out]
            n3590 = property on="XY Intensity Map" class="IntGraph (strict)"() -> ("Cursor.Cursor X"=w4427:dbl, "Cursor.Cursor Y"=w4425:dbl)  [unwired: 2 in, 2 out]
            n3591 = property class="Bool (strict)"(reference=w4437, "Value"=FALSE) -> ()  [unwired: 1 in, 2 out]
            n3592 = Multiply(x=w4427, y=1000.0) -> (x*y=w4434:dbl)
            n3593 = Multiply(x=w4425, y=1000.0) -> (x*y=w4429:dbl)
            n3594 = Round To Nearest(number=w4434) -> (nearest integer value=w4432:dbl)
            n3595 = Round To Nearest(number=w4429) -> (nearest integer value=w4431:dbl)
            n3596 = Divide(x=w4432, y=1000.0) -> (x/y=w4426:dbl)
            n3597 = Divide(x=w4431, y=1000.0) -> (x/y=w4424:dbl)
            n3598 = local write "Scan X Center (V)"(w4426) -> ()
            n3599 = local write "Scan Y Center (V)"(w4424) -> ()
          }
          event "Scan X Res. (V)", "Scan Y Res. (V)", "Scan X Tot. Length (V)", "Scan Y Tot. Length": Value Change {
            n3600 = event-data() -> ()  [unwired: 1 in, 6 out]
            n3601 = local read "Acq Time (ms)"() -> (w4441:dbl)
            n3602 = local read "Scan X Tot. Length (V)"() -> (w4452:dbl)
            n3603 = local read "Scan Y Res. (V)"() -> (w4448:dbl)
            n3604 = local read "Scan Y Tot. Length"() -> (w4447:dbl)
            n3605 = local read "Scan X Res. (V)"() -> (w4451:dbl)
            n3606 = Add(x=w4441, y=200.0) -> (x+y=w4439:dbl)
            n3607 = Divide(x=w4452, y=w4451) -> (x/y=w4450:dbl)
            n3608 = Divide(x=w4447, y=w4448) -> (x/y=w4449:dbl)
            n3609 = Divide(x=w4439, y=1000.0) -> (x/y=w4443:dbl)
            n3610 = Increment(x=w4450) -> (x+1=w4438:dbl)
            n3611 = Increment(x=w4449) -> (x+1=w4446:dbl)
            n3612 = local write "Scan Y Num. Pts"(w4446) -> ()
            n3613 = Multiply(x=w4438, y=w4446) -> (x*y=w4445:dbl)
            n3614 = local write "Scan X Num. Pts"(w4438) -> ()
            n3615 = Multiply(x=w4445, y=w4443) -> (x*y=w4442:dbl)
            n3616 = local write "Expected (s)"(w4442) -> ()
          }
          event "Shutter Ctrls", "KCubeSolenoidControl": Mouse Down {
            n3617 = event-data() -> ()  [unwired: 1 in, 8 out]
            n3618 = local read "KCube Shutter On?"() -> (w4453:bool)
            n3619 = control-ref of="Shutter Ctrls"() -> (w4455:refnum<vi>)
            n3620 = control-ref of="KCube Shutter Device Reference"() -> (w4454:refnum<vi>)